vi "HFRR ADV v040 new software.vi"() -> ()   [LabVIEW 2025] (continued)
          frame #0 {
            w818 = T19."Disabled and Grayed Out" ("Disabled")
            w819 = TRUE ("Heater Button")
            n785 = property on="Humidity" class="Bool (strict)"("DisabledEnum"=w818) -> ()  [unwired: 2 in, 2 out]
            n786 = property on="Heater Button" class="Bool (strict)"("DisabledEnum"=w818) -> ()  [unwired: 2 in, 2 out]
            n787 = local write "Heater Button"(w819) -> ()
            n788 = local write "Humidity"(w819) -> ()
            n789 = property on="Heater Button" class="Bool (strict)"("Val(Sgnl)"=TRUE ("Value (Signaling)")) -> ()  [unwired: 2 in, 2 out]
          }
          frame #1 {
            n790 = Wait (ms)(milliseconds to wait=u32 3000) -> ()  [unwired: 1 out]
          }
          frame #2 {
            n791 = local read "Set Temp"() -> (w825:dbl)
            n792 = Number To Fractional String(number=w825, precision (6)=i16 2) -> (F-format string=w822:string)  [unwired: 2 in]
            n793 = Concatenate Strings("ST;" ("Command"), w822) -> (w823:string)
            n794 = local write "Due Write"(w823) -> ()
          }
          frame #3 {
            n795 = Wait (ms)(milliseconds to wait=u32 1500) -> ()  [unwired: 1 out]
          }
          frame #4 {
            (unwired) i16 2 ("precision (6)")
            n796 = local read "WriteHumidity"() -> (w827:string[])
            n797 = local read "Set Rh"() -> (w830:dbl)
            n798 = Number To Fractional String(number=w830) -> (F-format string=w831:string)  [unwired: 3 in]
            n799 = Concatenate Strings("M;" ("new element/subarray"), w831) -> (w832:string)
            n800 = Insert Into Array(array=w827, new element=w832) -> (w828:string[])  [unwired: 1 in]
            n801 = local write "WriteHumidity"(w828) -> ()
            n802 = local write "Due Write"("HE;1" ("Command")) -> ()
          }
          frame #5 {
            n803 = Wait (ms)(milliseconds to wait=u32 1500) -> ()  [unwired: 1 out]
          }
          frame #6 {
            w835 = TRUE ("Reach point temp")
            n804 = local write "Reach point Humidity"(w835) -> ()
            n805 = local write "Reach point temp"(w835) -> ()
          }
        }
        n806 = local read "Auto Start Test"() -> (w815:bool)
        n807 = Not(x=w815) -> (.not. x?=w814:bool)
        n808 = Select(t=Auto_Start_enum."close", s=w814, f=w813) -> (s? t:f=w816:T15)
      }
      frame "Reach point" {
        w844 = TRUE ("PAUSE")
        w852 = 1.0 ("y")
        w855 = 1.0 ("y")
        n809 = local read "Set Temp"() -> (w837:dbl)
        n810 = local read "Set Humidity:"() -> (w851:dbl)
        n811 = local read "Humidity ( %RH )"() -> (w856:dbl)
        n812 = Add(x=w837, y=w855) -> (x+y=w854:dbl)
        n813 = Subtract(x=w837, y=w855) -> (x-y=w853:dbl)
        n814 = Add(x=w851, y=w852) -> (x+y=w850:dbl)
        n815 = Subtract(x=w851, y=w852) -> (x-y=w849:dbl)
        n816 = local read "TEMP"() -> (w857:dbl)
        n817 = In Range and Coerce(upper limit=w850, x=w856, lower limit=w849) -> (In Range?=w838:bool)  [unwired: 1 out]
        n818 = In Range and Coerce(upper limit=w854, x=w857, lower limit=w853) -> (In Range?=w839:bool)  [unwired: 1 out]
        n819 = case shown="True" w838 {
          frame False {
          }
          frame True {
            n820 = case shown="True" "Reach point Humidity" {
              selector: "Reach point Humidity" -> [_ w863]
              frame False {
              }
              frame True {
                n821 = local read "EVENT LOG"() -> (w860:string)
                n822 = Not(x=w863) -> (.not. x?=w862:bool)
                n823 = local write "Reach point Humidity"(w862) -> ()
                n824 = call "Event Log.vi"("Content"="Target Humidity reached", "EVENT LOG"=w860) -> ("EVENT LOG"=w861:string)  [unwired: 8 in, 1 out]
                n825 = local write "EVENT LOG"(w861) -> ()
              }
            }
          }
        }
        n826 = case shown="True" w839 {
          frame False {
          }
          frame True {
            n827 = case shown="True" "Reach point temp" {
              selector: "Reach point temp" -> [_ w869]
              frame False {
              }
              frame True {
                n828 = local read "EVENT LOG"() -> (w866:string)
                n829 = Not(x=w869) -> (.not. x?=w868:bool)
                n830 = local write "Reach point temp"(w868) -> ()
                n831 = call "Event Log.vi"("Content"="Target Temperature reached", "EVENT LOG"=w866) -> ("EVENT LOG"=w867:string)  [unwired: 8 in, 1 out]
                n832 = local write "EVENT LOG"(w867) -> ()
              }
            }
          }
        }
        n833 = local read "Auto Start Test"() -> (w842:bool)
        n834 = And(x=w839, y=w838) -> (x .and. y?=w848:bool)
        n835 = Select(t=Auto_Start_enum."Maintain Stage" ("Enum - Selector"), s=w848, f=Auto_Start_enum."Reach point" ("Enum - Selector")) -> (s? t:f=w845:T15)
        n836 = Not(x=w842) -> (.not. x?=w841:bool)
        n837 = Select(t=Auto_Start_enum."close", s=w841, f=w845) -> (s? t:f=w843:T15)
        n838 = call "ELAPSED TIMER VI.vi"("RESET"=w844, "PAUSE"=w844) -> ()  [unwired: 7 in, 3 out]
      }
      frame "Maintain Stage" {
        w884 = 2.0 ("y")
        w883 = 1.0 ("y")
        # "Humidity and  temperatures Set Point  have been reached"
        n839 = local read "Set Temp"() -> (w870:dbl)
        n840 = local read "Set Humidity:"() -> (w887:dbl)
        n841 = local read "Humidity ( %RH )"() -> (w890:dbl)
        n842 = Add(x=w870, y=w883) -> (x+y=w889:dbl)
        n843 = Subtract(x=w870, y=w883) -> (x-y=w888:dbl)
        n844 = local read "TEMP"() -> (w891:dbl)
        n845 = Add(x=w887, y=w884) -> (x+y=w886:dbl)
        n846 = Subtract(x=w887, y=w884) -> (x-y=w885:dbl)
        n847 = In Range and Coerce(upper limit=w889, x=w891, lower limit=w888) -> (In Range?=w882:bool)  [unwired: 1 out]
        n848 = In Range and Coerce(upper limit=w886, x=w890, lower limit=w885) -> (In Range?=w881:bool)  [unwired: 1 out]
        n849 = And(x=w882, y=w881) -> (x .and. y?=w880:bool)
        n850 = Not(x=w880) -> (.not. x?=w879:bool)
        n851 = call "ELAPSED TIMER VI.vi"("TARGET"=60.0, "RESET"=w879, "PAUSE"=FALSE) -> ("ELAPSED INDICATION"=w876:bool)  [unwired: 6 in, 2 out]
        n852 = case shown="True" w876 {
          tunnel: w876 -> [_ w894]
          tunnel: [Auto_Start_enum."Maintain Stage" ("Enum - Selector") w893] -> w874
          frame False {
          }
          frame True {
            n853 = stacked-sequence {
              tunnel: w894 -> [_ _ _ _ _]
              tunnel: [_ _ _ _ Auto_Start_enum."Start Stage" ("Enum - Selector")] -> w893
              frame #0 {
                n854 = local read "EVENT LOG"() -> (w896:string)
                n855 = call "Event Log.vi"("Content"="Humidity and temperature set point has stabilized.", "EVENT LOG"=w896) -> ("EVENT LOG"=w897:string)  [unwired: 8 in, 1 out]
                n856 = local write "EVENT LOG"(w897) -> ()
              }
              frame #1 {
                n857 = Wait (ms)(milliseconds to wait=u32 100) -> ()  [unwired: 1 out]
              }
              frame #2 {
                n858 = local read "EVENT LOG"() -> (w900:string)
                n859 = call "Event Log.vi"("Content"="Auto Test Started", "EVENT LOG"=w900) -> ("EVENT LOG"=w901:string)  [unwired: 8 in, 1 out]
                n860 = local write "EVENT LOG"(w901) -> ()
              }
              frame #3 {
                w902 = TRUE ("RUN")
                n861 = local write "RUN"(w902) -> ()
                n862 = property on="Auto Start Temp" class="Bool (strict)"("Val(Sgnl)"=w902) -> ()  [unwired: 2 in, 2 out]
                "Auto Start Temp" <- w902
              }
              frame #4 {
              }
            }
          }
        }
        n863 = local read "Auto Start Test"() -> (w873:bool)
        n864 = Not(x=w873) -> (.not. x?=w872:bool)
        n865 = Select(t=Auto_Start_enum."close", s=w872, f=w874) -> (s? t:f=w875:T15)
      }
      frame "Start Stage" {
        w904 = TRUE ("PAUSE")
        n866 = local read "Auto Start Test"() -> (w909:bool)
        n867 = Not(x=w909) -> (.not. x?=w908:bool)
        n868 = Select(t=Auto_Start_enum."close" ("Enum - Selector"), s=w908, f=Auto_Start_enum."Start Stage" ("Enum - Selector")) -> (s? t:f=w905:T15)
        n869 = call "ELAPSED TIMER VI.vi"("RESET"=w904, "PAUSE"=w904) -> ()  [unwired: 7 in, 3 out]
      }
      frame "close" {
        w911 = FALSE ("Heater Button")
        n870 = local write "RUN"(w911) -> ()
        n871 = local write "Heater Button"(w911) -> ()
        n872 = local write "Humidity"(w911) -> ()
        n873 = local write "Auto Start Test"(w911) -> ()
        n874 = property on="Heater Button" class="Bool (strict)"("Val(Sgnl)"=FALSE ("Value (Signaling)")) -> ()  [unwired: 2 in, 2 out]
      }
      frame "Exit" {
      }
    }
    n875 = Wait (ms)(milliseconds to wait=u32 100) -> ()  [unwired: 1 out]
    n876 = local read "Quit"() -> (w807:bool)
  }
  n877 = property on="Service Password Log" class="Str"("Visible"=w21) -> ()  [unwired: 2 in, 2 out]
  n878 = property on="Password 3" class="Clust (strict)"("Visible"=w21) -> ()  [unwired: 2 in, 2 out]
  n879 = while {
    stop <- w940 stop-if-true
    w923 = errorcluster {"status"=FALSE, "code"=0, "source"=""} ("error in (no error) 3")
    # "this loop is for manual report generation"
    n880 = local read "Confirm Measrurement"() -> (w922:bool)
    n881 = case shown="True" w922 {
      selector: w922 -> [_ w1030]
      tunnel: errorcluster {"status"=FALSE, "code"=0, "source"=""} ("error in (no error) 3") -> [_ w1031]
      tunnel: [_ w1029] -> _
      frame False {
      }
      frame True {
        n882 = stacked-sequence {
          tunnel: w1031 -> [_ w1069 _]
          tunnel: w1030 -> [_ _ w1180]
          tunnel: [_ w1058 _] -> w1029
          frame #0 {
            n883 = String To Path(string="C:\\LAB-IQ\\Image Calibrate v01.dcf") -> (path=w1034:path)
            n884 = Open/Create/Replace File ("Open File")(file path (use dialog)=w1034) -> (refnum out=w1035:refnum<file>)  [unwired: 5 in, 2 out]
            n885 = for {
              N: 4 -> [_]
              tunnel: w1035 -> [w1041]
              i -> [w1037]
              n886 = Read from Text File ("Read File")(file (use dialog)=w1041) -> (text=w1042:string)  [unwired: 3 in, 3 out]
              n887 = String Subset(string=w1042, offset (0)=6, length (rest)=10 ("length (rest)")) -> (substring=w1038:string)
              n888 = Fract/Exp String To Number(string=w1038) -> (number=w1036:dbl)  [unwired: 3 in, 1 out]
              n889 = case shown="3" w1037 {
                tunnel: w1036 -> [w1043 w1044 _ w1045 _]
                frame 0 {
                  n890 = local write "5x Gain"(w1043) -> ()
                }
                frame 1 {
                  n891 = local write "10x Gain"(w1044) -> ()
                }
                frame 2 {
                }
                frame 3 {
                  n892 = local write "100x gain"(w1045) -> ()
                }
                frame 4, Default {
                }
              }
            }
          }
          frame #1 {
            w1049 = "_5x" ("regular expression")
            n893 = local read "Image path  2"() -> (w1048:path)
            n894 = local read "TEST STANDARD"() -> (w1053:T3)
            n895 = Strip Path(path=w1048) -> (name=w1051:string)  [unwired: 1 out]
            n896 = case shown="\"ISO 12156\"" w1053 {
              tunnel: ["ASTM D6079" "ISO 12156"] -> w1052
              frame "ASTM D6079", Default {
              }
              frame "ISO 12156" {
              }
            }
            n897 = call "IMAGE ANALYSIS.vi"("Enum"=POST_ANALYSIS_ENUM."GET MEASUREMENTS", "error in"=w1069) -> ("error out"=w1076:errorcluster)  [unwired: 8 in, 1 out]
            n898 = Match Pattern(string=w1051, regular expression=w1049) -> (match substring=w1050:string)  [unwired: 1 in, 3 out]
            n899 = local read "Magnification :"() -> (w1062:string)
            n900 = Equal?(x=w1050, y=w1049) -> (x = y?=w1047:bool)
            n901 = call "Stall Data Flow.vim"("value in"=w1076, "milliseconds to wait"=u32 1000) -> ("value out"=w1075:errorcluster)  [unwired: 1 out]
            n902 = local read "Test File List :"() -> (w1073:string)
            n903 = case shown="False" w1047 {
              tunnel: [w1080 w1082] -> w1046
              frame False {
                n904 = local read "10x Gain"() -> (w1080:dbl)
                n905 = local write "Magnification :"("10x" ("Magnification :")) -> ()
              }
              frame True {
                n906 = local read "5x Gain"() -> (w1082:dbl)
                n907 = local write "Magnification :"("5x" ("Magnification :")) -> ()
              }
            }
            n908 = case shown="\"10x\"" w1062 {
              tunnel: [w1116 w1117] -> _
              frame "5x", Default {
                n909 = local read "5x Gain"() -> (w1116:dbl)
              }
              frame "10x" {
                # "5x"
                n910 = local read "10x Gain"() -> (w1117:dbl)
              }
            }
            n911 = call "IMAGE ANALYSIS.vi"("Enum"=POST_ANALYSIS_ENUM."READ", "error in"=w1075) -> ("error out"=w1072:errorcluster, "data out"=w1063:string)  [unwired: 8 in]
            n912 = Match Pattern(string=w1063, regular expression="\"type\": ") -> (after substring=w1067:string)  [unwired: 1 in, 3 out]
            n913 = call "IMAGE PATH CREATION PY.vi"("error in (no error)"=w1072, "File Name :"=w1073) -> ("error out"=w1071:errorcluster, "File Path"=w1060:path, "File Path String:"=w1055:string)  [unwired: 7 in]
            n914 = Match Pattern(string=w1067, regular expression=",") -> (before substring=w1054:string)  [unwired: 1 in, 3 out]
            n915 = local read "Calibration Tab"() -> (w1057:enum32{"Measrument", "Calibrate"})
            n916 = call "Stall Data Flow.vim"("value in"=w1071, "milliseconds to wait"=u32 250) -> ("value out"=w1056:errorcluster)  [unwired: 1 out]
            n917 = Equal?(x=w1054, y="\"rectangle\"") -> (x = y?=w1064:bool)
            n918 = case shown="False" w1064 {
              tunnel: w1063 -> [w1122 w1177]
              tunnel: w1046 -> [_ w1168]
              tunnel: cluster{"major":dbl, "minor":dbl, "average":dbl} {"major"=0.0, "minor"=0.0, "average"=0.0} -> [w1120 w1164]
              tunnel: [w1119 w1161] -> w1059
              tunnel: w1054 -> [w1121 _]
              tunnel: w1046 -> [w1118 _]
              frame False {
                n919 = Equal?(x=w1121, y="\"line\"") -> (x = y?=w1123:bool)
                n920 = case shown="True" w1123 {
                  tunnel: w1122 -> [_ w1138]
                  tunnel: w1120 -> [w1125 w1137]
                  tunnel: [w1125 w1135] -> w1119
                  tunnel: w1118 -> [_ w1134]
                  frame False {
                  }
                  frame True {
                    w1133 = 0.0 ("Major Axis")
                    n921 = Match Pattern(string=w1138, regular expression="\"length_px\":") -> (after substring=w1136:string)  [unwired: 1 in, 3 out]
                    n922 = property on="Major Axis" class="DigNum (strict)"("Caption.Text"="") -> ()  [unwired: 2 in, 2 out]
                    n923 = property on="Minor Axis" class="DigNum (strict)"("Caption.Text"="") -> ()  [unwired: 2 in, 2 out]
                    n924 = property on="Average" class="DigNum (strict)"("Caption.Text"="Line") -> ()  [unwired: 2 in, 2 out]
                    n925 = Fract/Exp String To Number(string=w1136, default (0 dbl)=0.0 ("default (0 DBL)")) -> (number=w1132:dbl)  [unwired: 2 in, 1 out]
                    "Pixel Value" <- w1132
                    n926 = Multiply(x=w1132, y=w1134) -> (x*y=w1145:dbl)
                    n927 = Multiply(x=w1145, y=1000.0) -> (x*y=w1128:dbl)
                    n928 = Divide(x=w1128, y=1000.0) -> (x/y=w1131:dbl)
                    n929 = local write "Measurment (mm)"(w1131) -> ()
                    n930 = Bundle By Name(cluster=w1137, "average"=w1128) -> (w1135:cluster{"major":dbl, "minor":dbl, "average":dbl})
                    n931 = Number To Fractional String(number=w1128, precision (6)=i16 1) -> (F-format string=w1127:string)  [unwired: 2 in]
                    n932 = local write "Minor Axis"(w1133) -> ()
                    n933 = local write "Major Axis"(w1133) -> ()
                    n934 = Fract/Exp String To Number(string=w1127) -> (number=w1126:dbl)  [unwired: 3 in, 1 out]
                    n935 = local write "Average"(w1126) -> ()
                  }
                }
              }
              frame True {
                w1165 = 1000.0 ("y")
                w1171 = 0.0 ("default (0 DBL)")
                n936 = Match Pattern(string=w1177, regular expression=" \"width_px\":") -> (after substring=w1175:string)  [unwired: 1 in, 3 out]
                n937 = Match Pattern(string=w1175, regular expression="\"height_px\":") -> (before substring=w1173:string, after substring=w1172:string)  [unwired: 1 in, 2 out]
                n938 = Fract/Exp String To Number(string=w1173, default (0 dbl)=w1171) -> (number=w1170:dbl)  [unwired: 2 in, 1 out]
                n939 = Fract/Exp String To Number(string=w1172, default (0 dbl)=w1171) -> (number=w1169:dbl)  [unwired: 2 in, 1 out]
                n940 = Multiply(x=w1170, y=w1168) -> (x*y=w1167:dbl)
                n941 = Multiply(x=w1169, y=w1168) -> (x*y=w1166:dbl)
                n942 = Multiply(x=w1167, y=w1165) -> (x*y=w1151:dbl)
                n943 = Multiply(x=w1166, y=w1165) -> (x*y=w1149:dbl)
                n944 = Add(x=w1151, y=w1149) -> (x+y=w1163:dbl)
                n945 = property on="Major Axis" class="DigNum (strict)"("Caption.Text"="Major Axis") -> ()  [unwired: 2 in, 2 out]
                n946 = property on="Minor Axis" class="DigNum (strict)"("Caption.Text"="Minor Axis") -> ()  [unwired: 2 in, 2 out]
                n947 = property on="Average" class="DigNum (strict)"("Caption.Text"="Average") -> ()  [unwired: 2 in, 2 out]
                n948 = Divide(x=w1163, y=2.0) -> (x/y=w1147:dbl)
                n949 = Bundle By Name(cluster=w1164, "major"=w1151, "minor"=w1149, "average"=w1147) -> (w1161:cluster{"major":dbl, "minor":dbl, "average":dbl})
                n950 = Number To Fractional String(number=w1149, precision (6)=i16 1) -> (F-format string=w1156:string)  [unwired: 2 in]
                n951 = Number To Fractional String(number=w1147, precision (6)=i16 1) -> (F-format string=w1157:string)  [unwired: 2 in]
                n952 = Number To Fractional String(number=w1151, precision (6)=i16 1) -> (F-format string=w1155:string)  [unwired: 2 in]
                n953 = Fract/Exp String To Number(string=w1156) -> (number=w1148:dbl)  [unwired: 3 in, 1 out]
                n954 = Fract/Exp String To Number(string=w1157) -> (number=w1146:dbl)  [unwired: 3 in, 1 out]
                n955 = Fract/Exp String To Number(string=w1155) -> (number=w1150:dbl)  [unwired: 3 in, 1 out]
                n956 = local write "Major Axis"(w1150) -> ()
                n957 = local write "Average"(w1146) -> ()
                n958 = local write "Minor Axis"(w1148) -> ()
              }
            }
            n959 = case shown="\"Measrument\", Default" w1057 {
              tunnel: w1060 -> [w1090 _]
              tunnel: w1059 -> [w1089 _]
              tunnel: [w1086 w1115] -> w1058
              tunnel: w1056 -> [w1088 w1115]
              tunnel: w1055 -> [w1087 _]
              tunnel: w1052 -> [w1085 _]
              frame "Measrument", Default {
                n960 = stacked-sequence {
                  tunnel: w1090 -> [w1108 _]
                  tunnel: w1089 -> [w1106 _]
                  tunnel: w1088 -> [w1104 _]
                  tunnel: w1087 -> [w1103 _]
                  tunnel: [w1098 _] -> w1086
                  tunnel: w1085 -> [w1091 _]
                  frame #0 {
                    n961 = call "IMAGE ANALYSIS.vi"("Enum"=POST_ANALYSIS_ENUM."SAVE IMAGE", "error in"=w1104, "IMAGE FILE PATH"=w1103) -> ("error out"=w1102:errorcluster)  [unwired: 7 in, 1 out]
                    n962 = call "Stall Data Flow.vim"("value in"=w1102, "milliseconds to wait"=u32 1000) -> ("value out"=w1093:errorcluster)  [unwired: 1 out]
                    n963 = local read "Test File List :"() -> (w1110:string)
                    n964 = call "IMAGE ANALYSIS.vi"("Enum"=POST_ANALYSIS_ENUM."MINIMIZE UI", "error in"=w1093) -> ("error out"=w1100:errorcluster)  [unwired: 8 in, 1 out]
                    n965 = Bundle By Name(cluster=T27 {"File Name"="", "Test Method"="", "Operator"="", "Fuel Description"="", "Date and time"=""} ("Main Ref"), "Test Method"=w1091, "File Name"=w1110) -> (w1111:T27)
                    n966 = call "Stall Data Flow.vim"("value in"=w1100, "milliseconds to wait"=u32 1500) -> ("value out"=w1095:errorcluster)  [unwired: 1 out]
                    n967 = call "duf file read.vi"("error in (no error)"=w1095, "Main Ref"=w1111) -> ("error out"=w1109:errorcluster, "Main Ref 2"=w1107:T27)  [unwired: 8 in]
                    n968 = call "DETECTION REPORT for manual.vi"("error in (no error)"=w1109, "return value 3"=w1106, "Image File Path"=w1108, "Main Ref"=w1107) -> ("error out"=w1105:errorcluster)  [unwired: 7 in]
                    n969 = call <vilib>:"Clear Errors.vi"("error in (no error)"=w1105) -> ("error out"=w1096:errorcluster)  [unwired: 5 in, 1 out]
                    n970 = call "IMAGE ANALYSIS.vi"("Enum"=POST_ANALYSIS_ENUM."MINIMIZE UI", "error in"=w1096) -> ("error out"=w1098:errorcluster)  [unwired: 8 in, 1 out]
                  }
                  frame #1 {
                    n971 = local write "Main Tab"(T2."HOME" ("Main Tab")) -> ()
                    n972 = local write "Main Dashboard Buttons"(T1."Home" ("Main Dashboard Buttons")) -> ()
                  }
                }
              }
              frame "Calibrate" {
              }
            }
          }
          frame #2 {
            n973 = Not(x=w1180) -> (.not. x?=w1179:bool)
            n974 = local write "Confirm Measrurement"(w1179) -> ()
            n975 = local read "Calibration Tab"() -> (w1178:enum32{"Measrument", "Calibrate"})
            n976 = case shown="\"Measrument\", Default" w1178 {
              frame "Measrument", Default {
                (unwired) T21."HOME" ("Main Tab")
                n977 = local write "Main Tab"(T2."HOME" ("Main Tab")) -> ()
              }
              frame "Calibrate" {
              }
            }
          }
        }
      }
    }
    n978 = local read "Humidity"() -> (w914:bool)
    n979 = local read "Save Change"() -> (w919:bool)
    n980 = local read "Calibrate"() -> (w920:bool)
    n981 = local read "Auto Start Test"() -> (w915:bool)
    n982 = case shown="True" w920 {
      selector: w920 -> [_ w1027]
      frame False {
      }
      frame True {
        n983 = Not(x=w1027) -> (.not. x?=w1026:bool)
        n984 = local write "Calibrate"(w1026) -> ()
        n985 = local write "Calibration Tab"(enum32{"Measrument", "Calibrate"}."Calibrate" ("Calibration Tab")) -> ()
      }
    }
    n986 = case shown="True" w919 {
      selector: w919 -> [_ w971]
      frame False {
      }
      frame True {
        n987 = stacked-sequence {
          tunnel: w971 -> [_ _ _ _ w1025]
          frame #0 {
            n988 = call "IMAGE ANALYSIS.vi"("Enum"=POST_ANALYSIS_ENUM."HIDE UI") -> ()  [unwired: 9 in, 2 out]
          }
          frame #1 {
            n989 = local read "100x gain"() -> (w973:dbl)
            n990 = local read "10x Gain"() -> (w974:dbl)
            n991 = local read "5x Gain"() -> (w975:dbl)
            n992 = Number To Fractional String(number=w974, width (-)=i16 4, precision (6)=i16 7) -> (F-format string=w996:string)  [unwired: 1 in]
            n993 = Number To Fractional String(number=0.0, width (-)=i16 4, precision (6)=i16 7) -> (F-format string=w991:string)  [unwired: 1 in]
            n994 = Number To Fractional String(number=w973, width (-)=i16 4, precision (6)=i16 7) -> (F-format string=w979:string)  [unwired: 1 in]
            n995 = Number To Fractional String(number=w975, width (-)=i16 10 ("precision (6)"), precision (6)=i16 7) -> (F-format string=w1005:string)  [unwired: 1 in]
            n996 = Concatenate Strings("[CH1]" ("string"), w1005, " - 5x Gain" ("string"), "\r") -> (w995:string)
            n997 = Concatenate Strings("[CH2]" ("string"), w996, " - 10x Gain" ("string"), "\r") -> (w994:string)
            n998 = Concatenate Strings("[CH3]" ("string"), w991, " - 20x Gain" ("string"), "\r") -> (w985:string)
            n999 = Concatenate Strings("[CH4]" ("string"), w979, " - 100x Gain" ("string"), "\r") -> (w978:string)
            n1000 = String To Path(string="C:\\LAB-IQ\\Image Calibrate v01.dcf") -> (path=w1008:path)
            n1001 = Concatenate Strings(w995, w994, w985, w978) -> (w993:string)
            n1002 = call <vilib>:"Write Characters To File.vi"("append to file? (new file:F)"=FALSE, "character string"=w993, "file path (dialog if empty)"=w1008) -> ()  [unwired: 2 in, 1 out]
          }
          frame #2 {
            n1003 = String To Path(string="C:\\LAB-IQ\\Image Calibrate v01.dcf") -> (path=w1011:path)
            n1004 = Open/Create/Replace File ("Open File")(file path (use dialog)=w1011) -> (refnum out=w1012:refnum<file>)  [unwired: 5 in, 2 out]
            n1005 = for {
              N: 4 -> [_]
              tunnel: w1012 -> [w1018]
              i -> [w1014]
              n1006 = Read from Text File ("Read File")(file (use dialog)=w1018) -> (text=w1019:string)  [unwired: 3 in, 3 out]
              n1007 = String Subset(string=w1019, offset (0)=6, length (rest)=10 ("length (rest)")) -> (substring=w1015:string)
              n1008 = Fract/Exp String To Number(string=w1015) -> (number=w1013:dbl)  [unwired: 3 in, 1 out]
              n1009 = case shown="3" w1014 {
                tunnel: w1013 -> [w1020 w1021 _ w1022 _]
                frame 0 {
                  n1010 = local write "5x Gain"(w1020) -> ()
                }
                frame 1 {
                  n1011 = local write "10x Gain"(w1021) -> ()
                }
                frame 2 {
                }
                frame 3 {
                  n1012 = local write "100x gain"(w1022) -> ()
                }
                frame 4, Default {
                }
              }
            }
          }
          frame #3 {
            n1013 = call "IMAGE ANALYSIS.vi"("Enum"=POST_ANALYSIS_ENUM."SHOW UI") -> ()  [unwired: 9 in, 2 out]
          }
          frame #4 {
            n1014 = Not(x=w1025) -> (.not. x?=w1024:bool)
            n1015 = local write "Save Change"(w1024) -> ()
          }
        }
      }
    }
    n1016 = case shown="False" w915 {
      tunnel: w914 -> [w941 _]
      frame False {
        n1017 = case shown="True" w941 {
          frame False {
          }
          frame True {
            n1018 = local read "Set Humidity:"() -> (w945:dbl)
            n1019 = local read "Set Humidity:"() -> (w948:dbl)
            n1020 = local read "Humidity ( %RH )"() -> (w949:dbl)
            n1021 = Subtract(x=w945, y=2.0) -> (x-y=w943:dbl)
            n1022 = Add(x=w948, y=2.0) -> (x+y=w944:dbl)
            n1023 = In Range and Coerce(upper limit=w944, x=w949, lower limit=w943) -> (In Range?=w942:bool)  [unwired: 1 out]
            n1024 = case shown="True" w942 {
              frame False {
              }
              frame True {
                n1025 = case shown="True" "Manual Humididty Reached" {
                  selector: "Manual Humididty Reached" -> [_ w952]
                  frame False {
                  }
                  frame True {
                    n1026 = Not(x=w952) -> (.not. x?=w951:bool)
                    n1027 = local write "Manual Humididty Reached"(w951) -> ()
                    n1028 = local read "EVENT LOG"() -> (w954:string)
                    n1029 = call "Event Log.vi"("Content"="Target Humidity reached", "EVENT LOG"=w954) -> ("EVENT LOG"=w953:string)  [unwired: 8 in, 1 out]
                    n1030 = local write "EVENT LOG"(w953) -> ()
                  }
                }
              }
            }
          }
        }
      }
      frame True {
        n1031 = local write "Manual Humididty Reached"(TRUE ("Manual Humididty Reached")) -> ()
      }
    }
    n1032 = Wait (ms)(milliseconds to wait=u32 250) -> ()  [unwired: 1 out]
    n1033 = local read "Cap Live Image"() -> (w935:bool)
    n1034 = local read "SCAR MEASURMENT"() -> (w938:enum32{"Auto Scar", "Manual Scar"})
    n1035 = Equal?(x=w938, y=enum32{"Auto Scar", "Manual Scar"}."Manual Scar" ("SCAR MEASURMENT")) -> (x = y?=w936:bool)
    n1036 = And(x=w936, y=w935) -> (x .and. y?=w934:bool)
    n1037 = case shown="True" w934 {
      selector: w934 -> [_ w1266]
      frame False {
      }
      frame True {
        n1038 = stacked-sequence {
          tunnel: [_ _ _ w1285 _] -> _
          tunnel: w1266 -> [_ _ _ _ w1292]
          frame #0 {
            w1267 = 0.0
            n1039 = local write "Major Axis"(w1267) -> ()
            n1040 = local write "Minor Axis"(w1267) -> ()
            n1041 = local write "Average"(w1267) -> ()
          }
          frame #1 {
            n1042 = call "CAMERA LIVE FEED FGV.vi"("Enum - Menu"=CAMERA_LIVE_FEED_ENUM."CAMERA MINIMIZE") -> ()  [unwired: 9 in, 2 out]
          }
          frame #2 {
            n1043 = local read "Magnification len live scar"() -> (w1270:string)
            n1044 = case shown="\"10x\", Default" w1270 {
              tunnel: ["_10x" "_5x"] -> w1269
              frame "10x", Default {
              }
              frame "5x" {
              }
            }
            n1045 = local read "FILE 3"() -> (w1277:string)
            n1046 = call <vilib>:"Trim Whitespace.vi"("string"="C:\\LAB-IQ\\images\\") -> ("trimmed string"=w1279:string)  [unwired: 1 in]
            n1047 = String To Path(string=w1279) -> (path=w1278:path)
            n1048 = Concatenate Strings(w1277, w1269, ".png" ("string")) -> (w1276:string)
            n1049 = Build Path(base path=w1278, name or relative path=w1276) -> (appended path=w1275:path)
            n1050 = Path To String(path=w1275) -> (string=w1274:string)
            n1051 = call "CAMERA LIVE FEED FGV.vi"("Enum - Menu"=CAMERA_LIVE_FEED_ENUM."CAMERA SAVE", "Image Path"=w1274) -> ("error out"=w1272:errorcluster)  [unwired: 8 in, 1 out]
            n1052 = case shown="No Error" w1272 {
              frame No Error {
                n1053 = One Button Dialog(message="Image saved successfully") -> ()  [unwired: 1 in, 1 out]
              }
              frame Error {
              }
            }
          }
          frame #3 {
            n1054 = call "LIST FILE NAMES.vi"() -> ("error out"=w1287:errorcluster, "filenames"=w1284:string[])  [unwired: 10 in]
            n1055 = call "IMAGE ANALYSIS.vi"("Enum"=POST_ANALYSIS_ENUM."SHOW UI", "error in"=w1287) -> ("error out"=w1285:errorcluster)  [unwired: 8 in, 1 out]
            n1056 = property on="Test File List :" class="CmbBox"("Strings[]"=w1284) -> ()  [unwired: 2 in, 2 out]
          }
          frame #4 {
            (unwired) T26."Report" ("Main Dashboard Buttons")
            (unwired) T28."Report" ("Main Dashboard Buttons")
            n1057 = Not(x=w1292) -> (.not. x?=w1291:bool)
            n1058 = local write "Zoom Factore"(0.0 ("Zoom Factore")) -> ()
            n1059 = local write "Cap Live Image"(w1291) -> ()
            n1060 = local write "Main Tab"(T2."Adv Scar Report" ("Main Tab")) -> ()
            n1061 = property on="Cap Live Image" class="Bool (strict)"("BoolText.Text"="Capture Image" ("Boolean Text.Text")) -> ()  [unwired: 2 in, 2 out]
            n1062 = local write "Main Dashboard Buttons"(T1."Report" ("Main Dashboard Buttons")) -> ()
          }
        }
      }
    }
    n1063 = local read "change Gain"() -> (w918:bool)
    n1064 = local read "Back Square"() -> (w917:bool)
    n1065 = case shown="True" w918 {
      selector: w918 -> [_ w962]
      frame False {
      }
      frame True {
        n1066 = stacked-sequence {
          tunnel: w962 -> [_ w970]
          frame #0 {
            n1067 = local read "Actual (µm)"() -> (w966:dbl)
            n1068 = local read "Pixel Value"() -> (w965:dbl)
            n1069 = local read "Magnification :"() -> (w964:string)
            n1070 = Divide(x=w966, y=w965) -> (x/y=w963:dbl)
            n1071 = case shown="\"10x\"" w964 {
              tunnel: w963 -> [w967 w968]
              frame "10x" {
                n1072 = local write "10x Gain"(w967) -> ()
              }
              frame "5x", Default {
                n1073 = local write "5x Gain"(w968) -> ()
              }
            }
          }
          frame #1 {
            n1074 = Not(x=w970) -> (.not. x?=w969:bool)
            n1075 = local write "change Gain"(w969) -> ()
          }
        }
      }
    }
    n1076 = case shown="True" w917 {
      selector: w917 -> [_ w960]
      frame False {
      }
      frame True {
        n1077 = Not(x=w960) -> (.not. x?=w959:bool)
        n1078 = local write "Back Square"(w959) -> ()
        n1079 = local write "Calibration Tab"(enum32{"Measrument", "Calibrate"}."Measrument" ("Calibration Tab")) -> ()
      }
    }
    n1080 = local read "Rectangle Tool"() -> (w929:bool)
    n1081 = local read "Clear ROI Tool"() -> (w928:bool)
    n1082 = local read "Open Image"() -> (w933:bool)
    n1083 = local read "line tool"() -> (w930:bool)
    n1084 = local read "OUT"() -> (w931:bool)
    n1085 = local read "In"() -> (w932:bool)
    n1086 = case shown="True" w933 {
      selector: w933 -> [_ w1252]
      tunnel: [w1243 w1254] -> _
      tunnel: w923 -> [w1243 w1253]
      frame False {
      }
      frame True {
        w1245 = "_5x" ("regular expression")
        n1087 = Not(x=w1252) -> (.not. x?=w1251:bool)
        n1088 = local write "Open Image"(w1251) -> ()
        n1089 = call "IMAGE ANALYSIS.vi"("Enum"=POST_ANALYSIS_ENUM."HIDE UI", "error in"=w1253) -> ("error out"=w1261:errorcluster)  [unwired: 8 in, 1 out]
        n1090 = call "File Dialog"("start path"=path "C:/LAB-IQ/images", "error in"=w1261) -> ("selected path"=w1250:path, "error out"=w1259:errorcluster)  [unwired: 10 in, 2 out]
        "Image path  2" <- w1250
        n1091 = call <vilib>:"Clear Errors.vi"("error in (no error)"=w1259) -> ("error out"=w1258:errorcluster)  [unwired: 5 in, 1 out]
        n1092 = call "IMAGE ANALYSIS.vi"("Enum"=POST_ANALYSIS_ENUM."OPEN FILE", "error in"=w1258, "File Path"=w1250) -> ("error out"=w1257:errorcluster)  [unwired: 7 in, 1 out]
        n1093 = call <vilib>:"Clear Errors.vi"("error in (no error)"=w1257) -> ("error out"=w1256:errorcluster)  [unwired: 5 in, 1 out]
        n1094 = call "IMAGE ANALYSIS.vi"("Enum"=POST_ANALYSIS_ENUM."SHOW UI", "error in"=w1256) -> ("error out"=w1254:errorcluster)  [unwired: 8 in, 1 out]
        n1095 = local write "Zoom Factore"(100.0 ("Zoom Factore")) -> ()
        n1096 = local read "Image path  2"() -> (w1246:path)
        n1097 = Strip Path(path=w1246) -> (name=w1248:string)  [unwired: 1 out]
        n1098 = Match Pattern(string=w1248, regular expression=w1245) -> (match substring=w1247:string)  [unwired: 1 in, 3 out]
        n1099 = Equal?(x=w1247, y=w1245) -> (x = y?=w1244:bool)
        n1100 = case shown="True" w1244 {
          frame False {
            n1101 = local write "Magnification :"("10x" ("Magnification :")) -> ()
          }
          frame True {
            n1102 = local write "Magnification :"("5x" ("Magnification :")) -> ()
          }
        }
      }
    }
    n1103 = case shown="True" w931 {
      selector: w931 -> [_ w1228]
      tunnel: w923 -> [w1225 w1233]
      tunnel: [w1225 w1227] -> _
      frame False {
      }
      frame True {
        n1104 = Not(x=w1228) -> (.not. x?=w1226:bool)
        n1105 = local read "Zoom Factore"() -> (w1231:dbl)
        n1106 = local write "OUT"(w1226) -> ()
        n1107 = call "IMAGE ANALYSIS.vi"("Enum"=POST_ANALYSIS_ENUM."ZOOM OUT", "error in"=w1233) -> ("error out"=w1227:errorcluster)  [unwired: 8 in, 1 out]
        n1108 = Divide(x=w1231, y=1.2) -> (x/y=w1229:dbl)
        n1109 = local write "Zoom Factore"(w1229) -> ()
      }
    }
    n1110 = case shown="True" w932 {
      selector: w932 -> [_ w1237]
      tunnel: w923 -> [w1234 w1242]
      tunnel: [w1234 w1235] -> _
      frame False {
      }
      frame True {
        n1111 = Not(x=w1237) -> (.not. x?=w1236:bool)
        n1112 = local read "Zoom Factore"() -> (w1240:dbl)
        n1113 = local write "In"(w1236) -> ()
        n1114 = call "IMAGE ANALYSIS.vi"("Enum"=POST_ANALYSIS_ENUM."ZOOM IN", "error in"=w1242) -> ("error out"=w1235:errorcluster)  [unwired: 8 in, 1 out]
        n1115 = Multiply(x=w1240, y=1.2) -> (x*y=w1238:dbl)
        n1116 = local write "Zoom Factore"(w1238) -> ()
      }
    }
    n1117 = case shown="True" w928 {
      selector: w928 -> [_ w1209]
      tunnel: w923 -> [w1207 w1211]
      tunnel: [w1207 w1210] -> _
      frame False {
      }
      frame True {
        n1118 = Not(x=w1209) -> (.not. x?=w1208:bool)
        n1119 = local write "Clear ROI Tool"(w1208) -> ()
        n1120 = call "IMAGE ANALYSIS.vi"("Enum"=POST_ANALYSIS_ENUM."CLEAR ROI", "error in"=w1211) -> ("error out"=w1210:errorcluster)  [unwired: 8 in, 1 out]
      }
    }
    n1121 = case shown="True" w930 {
      selector: w930 -> [_ w1221]
      tunnel: w923 -> [w1219 w1224]
      tunnel: [w1219 w1222] -> _
      frame False {
      }
      frame True {
        n1122 = Not(x=w1221) -> (.not. x?=w1220:bool)
        n1123 = local write "line tool"(w1220) -> ()
        n1124 = call "IMAGE ANALYSIS.vi"("Enum"=POST_ANALYSIS_ENUM."DRAW LINE", "error in"=w1224) -> ("error out"=w1222:errorcluster)  [unwired: 8 in, 1 out]
      }
    }
    n1125 = case shown="True" w929 {
      selector: w929 -> [_ w1215]
      tunnel: w923 -> [w1213 w1217]
      tunnel: [w1213 w1216] -> _
      frame False {
      }
      frame True {
        n1126 = Not(x=w1215) -> (.not. x?=w1214:bool)
        n1127 = local write "Rectangle Tool"(w1214) -> ()
        n1128 = call "IMAGE ANALYSIS.vi"("Enum"=POST_ANALYSIS_ENUM."DRAW REC", "error in"=w1217) -> ("error out"=w1216:errorcluster)  [unwired: 8 in, 1 out]
      }
    }
    n1129 = local read "SCAR MEASURMENT"() -> (w916:enum32{"Auto Scar", "Manual Scar"})
    n1130 = local read "Fit to Screen Tool"() -> (w925:bool)
    n1131 = local read "Resize Tool"() -> (w924:bool)
    n1132 = case shown="\"Manual Scar\", Default" w916 {
      frame "Auto Scar" {
        n1133 = property on="Cap Live Image" class="Bool (strict)"("BoolText.Text"="Report" ("Boolean Text.Text")) -> ()  [unwired: 2 in, 2 out]
      }
      frame "Manual Scar", Default {
        n1134 = property on="Cap Live Image" class="Bool (strict)"("BoolText.Text"="Save Image" ("Boolean Text.Text")) -> ()  [unwired: 2 in, 2 out]
      }
    }
    n1135 = local read "ROI Color Tool"() -> (w926:bool)
    n1136 = local read "Pan Tool"() -> (w927:bool)
    n1137 = case shown="True" w927 {
      selector: w927 -> [_ w1203]
      tunnel: w923 -> [w1201 w1205]
      tunnel: [w1201 w1204] -> _
      frame False {
      }
      frame True {
        n1138 = Not(x=w1203) -> (.not. x?=w1202:bool)
        n1139 = call "IMAGE ANALYSIS.vi"("Enum"=POST_ANALYSIS_ENUM."PAN", "error in"=w1205) -> ("error out"=w1204:errorcluster)  [unwired: 8 in, 1 out]
        n1140 = local write "Pan Tool"(w1202) -> ()
      }
    }
    n1141 = case shown="True" w924 {
      selector: w924 -> [_ w1187]
      tunnel: w923 -> [w1182 w1184]
      tunnel: [w1182 w1183] -> _
      frame False {
      }
      frame True {
        n1142 = Not(x=w1187) -> (.not. x?=w1186:bool)
        n1143 = local write "Resize Tool"(w1186) -> ()
        n1144 = call "IMAGE ANALYSIS.vi"("Enum"=POST_ANALYSIS_ENUM."RESIZE MODE", "error in"=w1184) -> ("error out"=w1183:errorcluster)  [unwired: 8 in, 1 out]
      }
    }
    n1145 = case shown="True" w925 {
      selector: w925 -> [_ w1192]
      tunnel: [w1188 w1193] -> _
      tunnel: w923 -> [w1188 w1191]
      frame False {
      }
      frame True {
        n1146 = Not(x=w1192) -> (.not. x?=w1190:bool)
        n1147 = local write "Zoom Factore"(100.0 ("Zoom Factore")) -> ()
        n1148 = local write "Fit to Screen Tool"(w1190) -> ()
        n1149 = call "IMAGE ANALYSIS.vi"("Enum"=POST_ANALYSIS_ENUM."FIT", "error in"=w1191) -> ("error out"=w1193:errorcluster)  [unwired: 8 in, 1 out]
      }
    }
    n1150 = case shown="True" w926 {
      selector: w926 -> [_ w1198]
      tunnel: [w1195 w1199] -> _
      tunnel: w923 -> [w1195 w1196]
      frame False {
      }
      frame True {
        n1151 = Not(x=w1198) -> (.not. x?=w1197:bool)
        n1152 = local write "ROI Color Tool"(w1197) -> ()
        n1153 = call "IMAGE ANALYSIS.vi"("Enum"=POST_ANALYSIS_ENUM."SET ROI COLOR", "error in"=w1196) -> ("error out"=w1199:errorcluster)  [unwired: 8 in, 1 out]
      }
    }
    n1154 = local read "Quit"() -> (w940:bool)
  }
  n1155 = while {
    stop <- w1294 stop-if-true
    n1156 = local read "Image Path"() -> (w1297:path)
    n1157 = local read "Print 3"() -> (w1300:bool)
    n1158 = Equal?(x=w1297, y=path "") -> (x = y?=w1296:bool)
    n1159 = Not(x=w1296) -> (.not. x?=w1295:bool)
    n1160 = property on="Print 3" class="Bool (strict)"("Visible"=w1295) -> ()  [unwired: 2 in, 2 out]
    n1161 = case shown="True" w1300 {
      frame False {
        n1162 = local write "Rd"(TRUE ("Boolean 7")) -> ()
      }
      frame True {
        n1163 = flat-sequence {
          tunnel: [w1340] -> w1308
          tunnel: [w1327] -> w1306
          tunnel: [w1337] -> w1302
          tunnel: w1308 -> [w1349]
          tunnel: [w1349] -> w1307
          tunnel: w1306 -> [w1348]
          tunnel: [w1348] -> w1305
          tunnel: [w1346] -> w1304
          tunnel: [w1345] -> w1303
          tunnel: w1302 -> [w1345]
          tunnel: w1307 -> [w1351]
          tunnel: w1305 -> [w1352]
          tunnel: w1304 -> [_]
          tunnel: w1303 -> [w1350]
          frame #0 {
            n1164 = case shown="True" "Rd" {
              frame False {
              }
              frame True {
                n1165 = while {
                  tunnel: "abcdefABCDEF" ("string 2") -> [w1319]
                  shift-right: [w1317] -> w1311
                  shift-left: "" -> [w1316]
                  i -> [w1326]
                  stop <- w1325 stop-if-true
                  n1166 = Random Number (0-1)() -> (number: 0 to 1=w1320:dbl)
                  n1167 = Multiply(x=w1320, y=62.0) -> (x*y=w1322:dbl)
                  n1168 = Decrement(x="Length 2") -> (x-1=w1315:i16)
                  n1169 = To Word Integer(number=w1322) -> (16bit integer=w1323:i16)
                  n1170 = String Subset(string=w1319, offset (0)=w1323, length (rest)=1 ("length (rest)")) -> (substring=w1318:string)
                  n1171 = Greater Or Equal?(x=w1326, y=w1315) -> (x >= y?=w1325:bool)
                  n1172 = Concatenate Strings(w1318, w1316) -> (w1317:string)
                }
                "String 10" <- w1311
                n1173 = local write "Rd"(FALSE ("Boolean 7")) -> ()
              }
            }
          }
          frame #1 {
            w1338 = "_resized.jpg" ("command line")
            (unwired) ".jpg -resize 320x240 " ("string")
            (unwired) "Choose an Image File" ("prompt")
            # "-resize 1798x425"
            n1174 = local read "Image Path"() -> (w1332:path)
            n1175 = Strip Path(path=w1332) -> (stripped path=w1327:path, name=w1328:string)
            n1176 = Match Pattern(string=w1328, regular expression=".jpg") -> (before substring=→"before substring 2":string, after substring=→"after substring":string)  [unwired: 1 in, 2 out]
            n1177 = Match Pattern(string=w1328, regular expression="\\") -> (before substring=w1334:string)  [unwired: 1 in, 3 out]
            n1178 = Match Pattern(string=w1334, regular expression=".jpg") -> (before substring=w1333:string)  [unwired: 1 in, 3 out]
            n1179 = Concatenate Strings("cmd /c convert " ("string"), w1333, ".jpg -resize 320x240  " ("command line"), w1333, w1338) -> (w1341:string)
            n1180 = call <vilib>:"System Exec.vi"("run minimized? (F)"=TRUE, "wait until completion? (T)"=TRUE, "working directory"=w1327, "command line"=w1341) -> ("error out"=w1340:errorcluster)  [unwired: 4 in, 3 out]
            "error out 2" <- w1340
            n1181 = Concatenate Strings(w1333, w1338) -> (w1337:string)
          }
          frame #2 {
            n1182 = Wait (ms)(milliseconds to wait=u32 2000 ("millisecond timer value")) -> (millisecond timer value=w1346:u32)
          }
          frame #3 {
            n1183 = case shown="No Error" w1351 {
              tunnel: w1352 -> [w1355 _]
              tunnel: w1350 -> [w1353 _]
              frame No Error {
                (unwired) ".jpg" ("string")
                n1184 = Path To String(path=w1355) -> (string=w1359:string)
                n1185 = Concatenate Strings(w1359, "\\" ("string"), w1353) -> (w1358:string)
                n1186 = String To Path(string=w1358) -> (path=w1357:path)
                n1187 = call <vilib>:"Read JPEG File.vi"("path to JPEG file"=w1357) -> ("image data"=w1361:T16)  [unwired: 8 in, 2 out]
                "image data" <- w1361
                n1188 = local write "Print 3"(FALSE ("Print 2")) -> ()
                n1189 = call <vilib>:"Draw Flattened Pixmap.vi"("image data"=w1361) -> ("new picture"=→"new picture":picture)  [unwired: 8 in]
              }
              frame Error {
              }
            }
          }
        }
      }
    }
    n1190 = Wait (ms)(milliseconds to wait=u32 20 ("millisecond timer value")) -> ()  [unwired: 1 out]
    n1191 = local read "Quit"() -> (w1294:bool)
  }
  n1192 = while {
    tunnel: w38 -> [_]
    tunnel: w24 -> [_]
    stop <- w1391 stop-if-true
    # "New Adv Logics"
    n1193 = local read "Main Tab"() -> (w1372:T2)
    n1194 = local read "Main Tab"() -> (w1389:T2)
    n1195 = local read "Sign In"() -> (w1388:bool)
    n1196 = case shown="\"Adv Scar\"" w1372 {
      frame "HOME", Default {
        n1197 = local read "LIVE FEED MIN TEMP"() -> (w1524:bool)
        n1198 = local write "LIVE FEED MAX TEMP"(TRUE ("LIVE FEED MAX TEMP")) -> ()
        n1199 = local read "CAMERA ROI MIN TEMP"() -> (w1522:bool)
        n1200 = case shown="True" w1524 {
          selector: w1524 -> [_ w1531]
          frame False {
          }
          frame True {
            n1201 = Not(x=w1531) -> (.not. x?=w1530:bool)
            n1202 = local write "LIVE FEED MIN TEMP"(w1530) -> ()
            n1203 = call "CAMERA LIVE FEED FGV.vi"("Enum - Menu"=CAMERA_LIVE_FEED_ENUM."CAMERA MINIMIZE") -> ()  [unwired: 9 in, 2 out]
          }
        }
        n1204 = case shown="True" w1522 {
          selector: w1522 -> [_ w1528]
          frame False {
          }
          frame True {
            n1205 = Not(x=w1528) -> (.not. x?=w1527:bool)
            n1206 = local write "CAMERA ROI MIN TEMP"(w1527) -> ()
            n1207 = call "IMAGE ANALYSIS.vi"("Enum"=POST_ANALYSIS_ENUM."MINIMIZE UI") -> ()  [unwired: 9 in, 2 out]
          }
        }
        n1208 = local write "CAMERA ROI MAX TEMP"(TRUE ("CAMERA ROI MAX TEMP")) -> ()
      }
      frame "Test Setup" {
        n1209 = local read "LIVE FEED MIN TEMP"() -> (w1534:bool)
        n1210 = local read "CAMERA ROI MIN TEMP"() -> (w1532:bool)
        n1211 = local write "LIVE FEED MAX TEMP"(TRUE ("LIVE FEED MAX TEMP")) -> ()
        n1212 = case shown="True" w1534 {
          selector: w1534 -> [_ w1541]
          frame False {
          }
          frame True {
            n1213 = Not(x=w1541) -> (.not. x?=w1540:bool)
            n1214 = local write "LIVE FEED MIN TEMP"(w1540) -> ()
            n1215 = call "CAMERA LIVE FEED FGV.vi"("Enum - Menu"=CAMERA_LIVE_FEED_ENUM."CAMERA MINIMIZE") -> ()  [unwired: 9 in, 2 out]
          }
        }
        n1216 = case shown="True" w1532 {
          selector: w1532 -> [_ w1538]
          frame False {
          }
          frame True {
            n1217 = Not(x=w1538) -> (.not. x?=w1537:bool)
            n1218 = local write "CAMERA ROI MIN TEMP"(w1537) -> ()
            n1219 = call "IMAGE ANALYSIS.vi"("Enum"=POST_ANALYSIS_ENUM."MINIMIZE UI") -> ()  [unwired: 9 in, 2 out]
          }
        }
        n1220 = local write "CAMERA ROI MAX TEMP"(TRUE ("CAMERA ROI MAX TEMP")) -> ()
      }
      frame "Acquire" {
        n1221 = local read "LIVE FEED MIN TEMP"() -> (w1544:bool)
        n1222 = local write "LIVE FEED MAX TEMP"(TRUE ("LIVE FEED MAX TEMP")) -> ()
        n1223 = local read "CAMERA ROI MIN TEMP"() -> (w1542:bool)
        n1224 = case shown="True" w1544 {
          selector: w1544 -> [_ w1551]
          frame False {
          }
          frame True {
            n1225 = Not(x=w1551) -> (.not. x?=w1550:bool)
            n1226 = local write "LIVE FEED MIN TEMP"(w1550) -> ()
            n1227 = call "CAMERA LIVE FEED FGV.vi"("Enum - Menu"=CAMERA_LIVE_FEED_ENUM."CAMERA MINIMIZE") -> ()  [unwired: 9 in, 2 out]
          }
        }
        n1228 = case shown="True" w1542 {
          selector: w1542 -> [_ w1548]
          frame False {
          }
          frame True {
            n1229 = Not(x=w1548) -> (.not. x?=w1547:bool)
            n1230 = local write "CAMERA ROI MIN TEMP"(w1547) -> ()
            n1231 = call "IMAGE ANALYSIS.vi"("Enum"=POST_ANALYSIS_ENUM."MINIMIZE UI") -> ()  [unwired: 9 in, 2 out]
          }
        }
        n1232 = local write "CAMERA ROI MAX TEMP"(TRUE ("CAMERA ROI MAX TEMP")) -> ()
      }
      frame "Adv Scar" {
        n1233 = local read "CAMERA ROI MIN TEMP"() -> (w1552:bool)
        n1234 = case shown="True" "LIVE FEED MAX TEMP" {
          selector: "LIVE FEED MAX TEMP" -> [_ w1573]
          frame False {
          }
          frame True {
            n1235 = Not(x=w1573) -> (.not. x?=w1572:bool)
            n1236 = local write "LIVE FEED MAX TEMP"(w1572) -> ()
            n1237 = call "CAMERA LIVE FEED FGV.vi"("Enum - Menu"=CAMERA_LIVE_FEED_ENUM."CAMERA RESTORE") -> ("error out"=w1563:errorcluster)  [unwired: 9 in, 1 out]
            n1238 = Type Cast(type=30, x=0) -> (*(type *) &x=w1567:i32)
            n1239 = Add(x=w1567, y=48) -> (x+y=w1568:i32)
            n1240 = call "CAMERA LIVE FEED FGV.vi"("Enum - Menu"=CAMERA_LIVE_FEED_ENUM."CAMERA MODE SET", "error in (no error)"=w1563, "CAMERA MODE"=w1568) -> ("error out"=w1560:errorcluster)  [unwired: 7 in, 1 out]
            n1241 = call "CAMERA LIVE FEED FGV.vi"("Enum - Menu"=CAMERA_LIVE_FEED_ENUM."CAMERA GRAY", "error in (no error)"=w1560) -> ("error out"=w1559:errorcluster)  [unwired: 8 in, 1 out]
            n1242 = call "LIST FILE NAMES.vi"("error in (no error)"=w1559) -> ("error out"=w1569:errorcluster, "filenames"=w1570:string[])  [unwired: 9 in]
            n1243 = property on="FILE 3" class="CmbBox"(error in=w1569, "Strings[]"=w1570) -> ()  [unwired: 1 in, 2 out]
          }
        }
        n1244 = case shown="True" w1552 {
          selector: w1552 -> [_ w1558]
          frame False {
          }
          frame True {
            n1245 = Not(x=w1558) -> (.not. x?=w1557:bool)
            n1246 = local write "CAMERA ROI MIN TEMP"(w1557) -> ()
            n1247 = call "IMAGE ANALYSIS.vi"("Enum"=POST_ANALYSIS_ENUM."MINIMIZE UI") -> ()  [unwired: 9 in, 2 out]
          }
        }
        n1248 = local write "CAMERA ROI MAX TEMP"(TRUE ("CAMERA ROI MAX TEMP")) -> ()
        "LIVE FEED MIN TEMP" <- TRUE ("LIVE FEED MIN TEMP")
      }
      frame "Adv Scar Report" {
        n1249 = local read "CAMERA ROI MAX TEMP"() -> (w1574:bool)
        n1250 = local read "LIVE FEED MIN TEMP"() -> (w1576:bool)
        n1251 = local write "LIVE FEED MAX TEMP"(TRUE ("LIVE FEED MAX TEMP")) -> ()
        n1252 = case shown="True" w1576 {
          selector: w1576 -> [_ w1585]
          frame False {
          }
          frame True {
            n1253 = Not(x=w1585) -> (.not. x?=w1584:bool)
            n1254 = local write "LIVE FEED MIN TEMP"(w1584) -> ()
            n1255 = call "CAMERA LIVE FEED FGV.vi"("Enum - Menu"=CAMERA_LIVE_FEED_ENUM."CAMERA MINIMIZE") -> ()  [unwired: 9 in, 2 out]
          }
        }
        n1256 = case shown="True" w1574 {
          selector: w1574 -> [_ w1582]
          frame False {
          }
          frame True {
            n1257 = Not(x=w1582) -> (.not. x?=w1580:bool)
            n1258 = local write "CAMERA ROI MAX TEMP"(w1580) -> ()
            n1259 = call "IMAGE ANALYSIS.vi"("Enum"=POST_ANALYSIS_ENUM."SHOW UI") -> ("error out"=w1579:errorcluster)  [unwired: 9 in, 1 out]
            n1260 = call "LIST FILE NAMES.vi"("error in (no error)"=w1579) -> ("filenames"=w1578:string[])  [unwired: 9 in, 1 out]
            n1261 = property on="Test File List :" class="CmbBox"("Strings[]"=w1578) -> ()  [unwired: 2 in, 2 out]
          }
        }
        n1262 = local write "CAMERA ROI MIN TEMP"(TRUE ("CAMERA ROI MIN TEMP")) -> ()
      }
      frame "Compare Files" {
        n1263 = local read "LIVE FEED MIN TEMP"() -> (w1588:bool)
        n1264 = local write "LIVE FEED MAX TEMP"(TRUE ("LIVE FEED MAX TEMP")) -> ()
        n1265 = local read "CAMERA ROI MIN TEMP"() -> (w1586:bool)
        n1266 = case shown="True" w1588 {
          selector: w1588 -> [_ w1595]
          frame False {
          }
          frame True {
            n1267 = Not(x=w1595) -> (.not. x?=w1594:bool)
            n1268 = local write "LIVE FEED MIN TEMP"(w1594) -> ()
            n1269 = call "CAMERA LIVE FEED FGV.vi"("Enum - Menu"=CAMERA_LIVE_FEED_ENUM."CAMERA MINIMIZE") -> ()  [unwired: 9 in, 2 out]
          }
        }
        n1270 = case shown="True" w1586 {
          selector: w1586 -> [_ w1592]
          frame False {
          }
          frame True {
            n1271 = Not(x=w1592) -> (.not. x?=w1591:bool)
            n1272 = local write "CAMERA ROI MIN TEMP"(w1591) -> ()
            n1273 = call "IMAGE ANALYSIS.vi"("Enum"=POST_ANALYSIS_ENUM."MINIMIZE UI") -> ()  [unwired: 9 in, 2 out]
          }
        }
        n1274 = local write "CAMERA ROI MAX TEMP"(TRUE ("CAMERA ROI MAX TEMP")) -> ()
      }
      frame "About" {
        n1275 = local read "LIVE FEED MIN TEMP"() -> (w1598:bool)
        n1276 = local write "LIVE FEED MAX TEMP"(TRUE ("LIVE FEED MAX TEMP")) -> ()
        n1277 = local read "CAMERA ROI MIN TEMP"() -> (w1597:bool)
        n1278 = case shown="True" w1598 {
          selector: w1598 -> [_ w1605]
          frame False {
          }
          frame True {
            n1279 = Not(x=w1605) -> (.not. x?=w1604:bool)
            n1280 = local write "LIVE FEED MIN TEMP"(w1604) -> ()
            n1281 = call "CAMERA LIVE FEED FGV.vi"("Enum - Menu"=CAMERA_LIVE_FEED_ENUM."CAMERA MINIMIZE") -> ()  [unwired: 9 in, 2 out]
          }
        }
        n1282 = case shown="True" w1597 {
          selector: w1597 -> [_ w1602]
          frame False {
          }
          frame True {
            n1283 = Not(x=w1602) -> (.not. x?=w1601:bool)
            n1284 = local write "CAMERA ROI MIN TEMP"(w1601) -> ()
            n1285 = call "IMAGE ANALYSIS.vi"("Enum"=POST_ANALYSIS_ENUM."MINIMIZE UI") -> ()  [unwired: 9 in, 2 out]
          }
        }
        n1286 = local write "CAMERA ROI MAX TEMP"(TRUE ("CAMERA ROI MIN TEMP")) -> ()
      }
      frame "Advance" {
        n1287 = local read "LIVE FEED MIN TEMP"() -> (w1608:bool)
        n1288 = local write "LIVE FEED MAX TEMP"(TRUE ("LIVE FEED MAX TEMP")) -> ()
        n1289 = local read "CAMERA ROI MIN TEMP"() -> (w1606:bool)
        n1290 = case shown="True" w1608 {
          selector: w1608 -> [_ w1615]
          frame False {
          }
          frame True {
            n1291 = Not(x=w1615) -> (.not. x?=w1614:bool)
            n1292 = local write "LIVE FEED MIN TEMP"(w1614) -> ()
            n1293 = call "CAMERA LIVE FEED FGV.vi"("Enum - Menu"=CAMERA_LIVE_FEED_ENUM."CAMERA MINIMIZE") -> ()  [unwired: 9 in, 2 out]
          }
        }
        n1294 = local write "CAMERA ROI MAX TEMP"(TRUE ("CAMERA ROI MAX TEMP")) -> ()
        n1295 = case shown="True" w1606 {
          selector: w1606 -> [_ w1612]
          frame False {
          }
          frame True {
            n1296 = Not(x=w1612) -> (.not. x?=w1611:bool)
            n1297 = local write "CAMERA ROI MIN TEMP"(w1611) -> ()
            n1298 = call "IMAGE ANALYSIS.vi"("Enum"=POST_ANALYSIS_ENUM."MINIMIZE UI") -> ()  [unwired: 9 in, 2 out]
          }
        }
      }
      frame "Mooha" {
        n1299 = local read "LIVE FEED MIN TEMP"() -> (w1618:bool)
        n1300 = local write "LIVE FEED MAX TEMP"(TRUE ("LIVE FEED MAX TEMP")) -> ()
        n1301 = local read "CAMERA ROI MIN TEMP"() -> (w1616:bool)
        n1302 = case shown="True" w1618 {
          selector: w1618 -> [_ w1625]